vi "Dresden R2R Sputter 03.02.2018 IY24.vi"() -> ()   [LabVIEW 2009] (continued)
                        n14329 = while {
                          i -> [w20883]
                          stop <- w20884 stop-if-true
                          n14330 = Greater?(x=w20883, y=50) -> (0:w20881:bool)
                          n14331 = local read "Cnt_Left_slow_di"() -> (w20887:bool)
                          n14332 = case shown="True" w20881 {
                            frame #0 {
                            }
                            frame #1 {
                              n14333 = local write "Semi"(TRUE ("Semi")) -> ()
                              n14334 = local write "Error Message"("Transfer process was\ncancelled.Please check left slow sensor." ("Error Message")) -> ()
                            }
                          }
                          n14335 = case shown="False" w20887 {
                            tunnel: [FALSE ("Ch1_pet_cool_up_do") TRUE ("Ch1_pet_cool_up_do")] -> w20886
                            frame #0 {
                              n14336 = Wait Until Next ms Multiple(millisecond multiple=u32 200) -> ()  [unwired: 1 out]
                              n14337 = local write "Cnt_Left_slow_do"(TRUE ("Ch1_pet_cool_up_do")) -> ()
                            }
                            frame #1 {
                            }
                          }
                          n14338 = local read "Semi"() -> (w20885:bool)
                          n14339 = Or(x=w20886, y=w20885) -> (x .or. y?=w20884:bool)
                        }
                      }
                      frame #1 {
                      }
                    }
                  }
                  frame #3 {
                    n14340 = local read "Semi"() -> (w20894:bool)
                    n14341 = case shown="False" w20894 {
                      frame #0 {
                        n14342 = while {
                          i -> [w20897]
                          stop <- w20898 stop-if-true
                          n14343 = Greater?(x=w20897, y=50) -> (0:w20895:bool)
                          n14344 = local read "Cnt_Left_limit_di"() -> (w20901:bool)
                          n14345 = case shown="True" w20895 {
                            frame #0 {
                            }
                            frame #1 {
                              n14346 = local write "Semi"(TRUE ("Semi")) -> ()
                              n14347 = local write "Error Message"("Transfer process was\ncancelled.Please check left limit sensor." ("Error Message")) -> ()
                            }
                          }
                          n14348 = case shown="False" w20901 {
                            tunnel: [FALSE ("Ch1_pet_cool_up_do") TRUE ("Ch1_pet_cool_up_do")] -> w20900
                            frame #0 {
                              n14349 = Wait Until Next ms Multiple(millisecond multiple=u32 200) -> ()  [unwired: 1 out]
                              n14350 = local write "Cnt_Left_limit_do"(TRUE ("Ch1_pet_cool_up_do")) -> ()
                            }
                            frame #1 {
                            }
                          }
                          n14351 = local read "Semi"() -> (w20899:bool)
                          n14352 = Or(x=w20900, y=w20899) -> (x .or. y?=w20898:bool)
                        }
                      }
                      frame #1 {
                      }
                    }
                  }
                  frame #4 {
                    n14353 = local read "Semi"() -> (w20908:bool)
                    n14354 = case shown="False" w20908 {
                      frame #0 {
                        n14355 = local write "CH1_2trns_18"(TRUE ("CH1_2trns_7")) -> ()
                        n14356 = Wait (ms)(milliseconds to wait=u32 500) -> ()  [unwired: 1 out]
                      }
                      frame #1 {
                      }
                    }
                  }
                }
              }
              frame #1 {
              }
            }
          }
          frame #20 {
            n14357 = local read "Semi"() -> (w20911:bool)
            n14358 = case shown="False" w20911 {
              frame #0 {
                n14359 = local write "CH1_2trns_19"(TRUE ("CH1_2trns_18")) -> ()
                n14360 = local write "Cnt_Do_Buzzer"(TRUE ("Transfer_ch1_2")) -> ()
                n14361 = Wait (ms)(milliseconds to wait=u32 1500) -> ()  [unwired: 1 out]
              }
              frame #1 {
              }
            }
          }
          frame #21 {
            n14362 = local read "Semi"() -> (w20915:bool)
            n14363 = case shown="False" w20915 {
              frame #0 {
                n14364 = local write "ch_present_position"(4.0 ("ch_present_position")) -> ()
                n14365 = local write "Transfer_ch3_4"(FALSE ("Transfer_ch1_2")) -> ()
                n14366 = local write "Cnt_Do_Buzzer"(FALSE ("Transfer_ch1_2")) -> ()
                n14367 = Wait (ms)(milliseconds to wait=u32 500) -> ()  [unwired: 1 out]
              }
              frame #1 {
              }
            }
          }
        }
      }
      frame #6 {
        n14368 = stacked-sequence {
          frame #0 {
            n14369 = Wait (ms)(milliseconds to wait=u32 1500) -> ()  [unwired: 1 out]
            n14370 = local write "Clean_trnsfr_4_3"(TRUE ("Clean_trnsfr_1_2")) -> ()
            n14371 = local write "system_status"("Chamber 4 to Chamber 3 Transfer Process in Progress." ("system_status")) -> ()
            n14372 = local write "final_process_messages"("Chamber 4 to Chamber 3  Transfer Process was completed." ("final_process_messages")) -> ()
          }
          frame #1 {
            n14373 = stacked-sequence {
              frame #0 {
                n14374 = local write "Routine_check_transfer"(TRUE ("Routine_check_transfer")) -> ()
                n14375 = Wait (ms)(milliseconds to wait=u32 100) -> ()  [unwired: 1 out]
              }
              frame #1 {
                n14376 = while {
                  i -> [w20933]
                  stop <- w20929 stop-if-true
                  n14377 = Greater Or Equal?(x=w20933, y=1500) -> (x >= y?=w20930:bool)
                  n14378 = Wait Until Next ms Multiple(millisecond multiple=u32 200) -> ()  [unwired: 1 out]
                  n14379 = case shown="True" w20930 {
                    frame #0 {
                    }
                    frame #1 {
                      # "Hata mesajı"
                      n14380 = local write "Semi"(TRUE ("Semi")) -> ()
                    }
                  }
                  n14381 = local read "Routine_check_transfer"() -> (w20926:bool)
                  n14382 = local read "Semi"() -> (w20928:bool)
                  n14383 = Not(x=w20926) -> (.not. x?=w20927:bool)
                  n14384 = Or(x=w20927, y=w20928) -> (x .or. y?=w20929:bool)
                }
              }
              frame #2 {
                n14385 = Wait (ms)(milliseconds to wait=u32 500) -> ()  [unwired: 1 out]
              }
            }
          }
          frame #2 {
            # "STARTED UP CH3"
            n14386 = disable-structure shown="Disabled" {
              frame #0 {
                n14387 = local read "Semi"() -> (w20936:bool)
                n14388 = case shown="False" w20936 {
                  frame #0 {
                    n14389 = local read "started_up_ch3"() -> (w20937:bool)
                    n14390 = case shown="False" w20937 {
                      frame #0 {
                        n14391 = stacked-sequence {
                          frame #0 {
                            n14392 = local read "Semi"() -> (w20938:bool)
                            n14393 = case shown="False" w20938 {
                              frame #0 {
                                n14394 = local write "Start_up_ch3"(TRUE ("Start_up_ch2")) -> ()
                              }
                              frame #1 {
                              }
                            }
                          }
                          frame #1 {
                            n14395 = local read "Semi"() -> (w20940:bool)
                            n14396 = case shown="False" w20940 {
                              frame #0 {
                                n14397 = Wait (ms)(milliseconds to wait=u32 16000) -> ()  [unwired: 1 out]
                              }
                              frame #1 {
                              }
                            }
                          }
                          frame #2 {
                            n14398 = local read "Semi"() -> (w20942:bool)
                            n14399 = case shown="False" w20942 {
                              frame #0 {
                                n14400 = while {
                                i -> [w20947]
                                stop <- w20944 stop-if-true
                                n14401 = Greater?(x=w20947, y=80) -> (0:w20945:bool)
                                n14402 = local read "started_up_ch3"() -> (w20943:bool)
                                n14403 = case shown="True" w20945 {
                                frame #0 {
                                }
                                frame #1 {
                                n14404 = local write "Semi"(TRUE ("Semi")) -> ()
                                n14405 = local write "Error Message"("Chamber 1 Pressure is not suitable  \nfor transfer process!\nPlease check connections." ("Error Message")) -> ()
                                }
                                }
                                n14406 = case shown="False" w20943 {
                                tunnel: [FALSE TRUE] -> w20944
                                frame #0 {
                                n14407 = Wait Until Next ms Multiple(millisecond multiple=u32 200) -> ()  [unwired: 1 out]
                                }
                                frame #1 {
                                }
                                }
                                }
                              }
                              frame #1 {
                              }
                            }
                          }
                          frame #3 {
                            n14408 = local read "Semi"() -> (w20953:bool)
                            n14409 = case shown="False" w20953 {
                              frame #0 {
                                n14410 = local write "CH1_2_trns_0"(TRUE ("CH1_2_trns_0")) -> ()
                                n14411 = Wait (ms)(milliseconds to wait=u32 1000) -> ()  [unwired: 1 out]
                              }
                              frame #1 {
                              }
                            }
                          }
                        }
                      }
                      frame #1 {
                      }
                    }
                  }
                  frame #1 {
                  }
                }
              }
              frame #1 {
              }
            }
          }
          frame #3 {
            # "STARTED UP CH2"
            n14412 = disable-structure shown="Disabled" {
              frame #0 {
                n14413 = local read "Semi"() -> (w20956:bool)
                n14414 = case shown="False" w20956 {
                  frame #0 {
                    n14415 = local read "started_up_ch2"() -> (w20957:bool)
                    n14416 = case shown="False" w20957 {
                      frame #0 {
                        n14417 = stacked-sequence {
                          frame #0 {
                            n14418 = local read "Semi"() -> (w20958:bool)
                            n14419 = case shown="False" w20958 {
                              frame #0 {
                                n14420 = local write "Start_up_ch2"(TRUE ("Start_up_ch2")) -> ()
                              }
                              frame #1 {
                              }
                            }
                          }
                          frame #1 {
                            n14421 = local read "Semi"() -> (w20960:bool)
                            n14422 = case shown="False" w20960 {
                              frame #0 {
                                n14423 = Wait (ms)(milliseconds to wait=u32 18000) -> ()  [unwired: 1 out]
                              }
                              frame #1 {
                              }
                            }
                          }
                          frame #2 {
                            n14424 = local read "Semi"() -> (w20962:bool)
                            n14425 = case shown="False" w20962 {
                              frame #0 {
                                n14426 = while {
                                i -> [w20967]
                                stop <- w20964 stop-if-true
                                n14427 = Greater?(x=w20967, y=90) -> (0:w20965:bool)
                                n14428 = local read "started_up_ch2"() -> (w20963:bool)
                                n14429 = case shown="True" w20965 {
                                frame #0 {
                                }
                                frame #1 {
                                n14430 = local write "Semi"(TRUE ("Semi")) -> ()
                                n14431 = local write "Error Message"("Chamber 2 Pressure is not suitable  \nfor transfer process!\nPlease check connections." ("Error Message")) -> ()
                                }
                                }
                                n14432 = case shown="False" w20963 {
                                tunnel: [FALSE TRUE] -> w20964
                                frame #0 {
                                n14433 = Wait Until Next ms Multiple(millisecond multiple=u32 200) -> ()  [unwired: 1 out]
                                }
                                frame #1 {
                                }
                                }
                                }
                              }
                              frame #1 {
                              }
                            }
                          }
                          frame #3 {
                            n14434 = local read "Semi"() -> (w20973:bool)
                            n14435 = case shown="False" w20973 {
                              frame #0 {
                                n14436 = local write "CH1_2_trns_1"(TRUE ("CH1_2_trns_0")) -> ()
                                n14437 = Wait (ms)(milliseconds to wait=u32 1000) -> ()  [unwired: 1 out]
                              }
                              frame #1 {
                              }
                            }
                          }
                        }
                      }
                      frame #1 {
                      }
                    }
                  }
                  frame #1 {
                  }
                }
              }
              frame #1 {
              }
            }
          }
          frame #4 {
            # "TRNS GV-BP OPEN"
            n14438 = local read "Semi"() -> (w20976:bool)
            n14439 = case shown="False" w20976 {
              frame #0 {
                n14440 = stacked-sequence {
                  frame #0 {
                    n14441 = local read "Semi"() -> (w20977:bool)
                    n14442 = case shown="False" w20977 {
                      frame #0 {
                        n14443 = while {
                          i -> [w20984]
                          stop <- w20979 stop-if-true
                          n14444 = Greater?(x=w20984, y=50) -> (0:w20982:bool)
                          n14445 = local read "Ch3_Trns_gv_bp2_di"() -> (w20978:bool)
                          n14446 = case shown="True" w20982 {
                            frame #0 {
                            }
                            frame #1 {
                              n14447 = local write "Semi"(TRUE ("Semi")) -> ()
                              n14448 = local write "Error Message"("Transfer process was cancelled.\nPlease check CH1-Trns-GV connections." ("Error Message")) -> ()
                            }
                          }
                          n14449 = case shown="False" w20978 {
                            tunnel: [FALSE TRUE] -> w20981
                            frame #0 {
                              n14450 = Wait Until Next ms Multiple(millisecond multiple=u32 200) -> ()  [unwired: 1 out]
                              n14451 = local write "Ch3_Trns_gv_bp2_do"(TRUE ("Ch1_pet_cool_up_do")) -> ()
                            }
                            frame #1 {
                            }
                          }
                          n14452 = local read "Semi"() -> (w20980:bool)
                          n14453 = Or(x=w20981, y=w20980) -> (x .or. y?=w20979:bool)
                        }
                      }
                      frame #1 {
                      }
                    }
                  }
                  frame #1 {
                    n14454 = local read "Semi"() -> (w20991:bool)
                    n14455 = case shown="False" w20991 {
                      frame #0 {
                        n14456 = Wait (ms)(milliseconds to wait=u32 500) -> ()  [unwired: 1 out]
                      }
                      frame #1 {
                      }
                    }
                  }
                  frame #2 {
                    n14457 = local read "Semi"() -> (w20993:bool)
                    n14458 = case shown="False" w20993 {
                      frame #0 {
                        n14459 = while {
                          i -> [w21000]
                          stop <- w20995 stop-if-true
                          n14460 = Greater?(x=w21000, y=50) -> (0:w20998:bool)
                          n14461 = local read "Ch4_Trns_gv_bp_di"() -> (w20994:bool)
                          n14462 = case shown="True" w20998 {
                            frame #0 {
                            }
                            frame #1 {
                              n14463 = local write "Semi"(TRUE ("Semi")) -> ()
                              n14464 = local write "Error Message"("Transfer process was cancelled.\nPlease check CH1-Trns-GV connections." ("Error Message")) -> ()
                            }
                          }
                          n14465 = case shown="False" w20994 {
                            tunnel: [FALSE TRUE] -> w20997
                            frame #0 {
                              n14466 = local write "Ch4_Trns_gv_bp_do"(TRUE ("Ch1_pet_cool_up_do")) -> ()
                              n14467 = Wait Until Next ms Multiple(millisecond multiple=u32 200) -> ()  [unwired: 1 out]
                            }
                            frame #1 {
                            }
                          }
                          n14468 = local read "Semi"() -> (w20996:bool)
                          n14469 = Or(x=w20997, y=w20996) -> (x .or. y?=w20995:bool)
                        }
                      }
                      frame #1 {
                      }
                    }
                  }
                  frame #3 {
                    n14470 = local read "Semi"() -> (w21007:bool)
                    n14471 = case shown="False" w21007 {
                      frame #0 {
                        n14472 = Wait (ms)(milliseconds to wait=u32 500) -> ()  [unwired: 1 out]
                      }
                      frame #1 {
                      }
                    }
                  }
                }
              }
              frame #1 {
              }
            }
          }
          frame #5 {
            # "TRNS GV OPEN"
            n14473 = local read "Semi"() -> (w21009:bool)
            n14474 = case shown="False" w21009 {
              frame #0 {
                n14475 = stacked-sequence {
                  frame #0 {
                    n14476 = local read "Semi"() -> (w21010:bool)
                    n14477 = case shown="False" w21010 {
                      frame #0 {
                        n14478 = local write "Ch3_Trns_gv_close_do"(FALSE ("Ch1_pet_cool_up_do")) -> ()
                      }
                      frame #1 {
                      }
                    }
                  }
                  frame #1 {
                    n14479 = local read "Semi"() -> (w21012:bool)
                    n14480 = case shown="False" w21012 {
                      frame #0 {
                        n14481 = while {
                          i -> [w21019]
                          stop <- w21014 stop-if-true
                          n14482 = Greater?(x=w21019, y=500) -> (0:w21017:bool)
                          n14483 = local read "Ch3_Trns_gv_open_di"() -> (w21013:bool)
                          n14484 = case shown="True" w21017 {
                            frame #0 {
                            }
                            frame #1 {
                              n14485 = local write "Semi"(TRUE ("Semi")) -> ()
                              n14486 = local write "Error Message"("Transfer process was cancelled.\nPlease check CH1-Trns-GV connections." ("Error Message")) -> ()
                            }
                          }
                          n14487 = case shown="False" w21013 {
                            tunnel: [FALSE TRUE] -> w21016
                            frame #0 {
                              n14488 = Wait Until Next ms Multiple(millisecond multiple=u32 200) -> ()  [unwired: 1 out]
                              n14489 = local write "Ch3_Trns_gv_open_do"(TRUE ("Ch1_pet_cool_up_do")) -> ()
                            }
                            frame #1 {
                            }
                          }
                          n14490 = local read "Semi"() -> (w21015:bool)
                          n14491 = Or(x=w21016, y=w21015) -> (x .or. y?=w21014:bool)
                        }
                      }
                      frame #1 {
                      }
                    }
                  }
                  frame #2 {
                    n14492 = local read "Semi"() -> (w21026:bool)
                    n14493 = case shown="False" w21026 {
                      frame #0 {
                        n14494 = local write "CH1_2trns_2"(TRUE ("CH1_2trns_5")) -> ()
                        n14495 = Wait (ms)(milliseconds to wait=u32 500) -> ()  [unwired: 1 out]
                      }
                      frame #1 {
                      }
                    }
                  }
                }
              }
              frame #1 {
              }
            }
          }
          frame #6 {
            # "TRNS GV control Trnsgv 2_3"
            n14496 = local read "Semi"() -> (w21029:bool)
            n14497 = case shown="False" w21029 {
              frame #0 {
                n14498 = stacked-sequence {
                  frame #0 {
                    n14499 = local read "Semi"() -> (w21030:bool)
                    n14500 = case shown="False" w21030 {
                      frame #0 {
                        n14501 = while {
                          i -> [w21037]
                          stop <- w21032 stop-if-true
                          n14502 = Greater?(x=w21037, y=50) -> (0:w21035:bool)
                          n14503 = local read "Ch3_TGV_control_di"() -> (w21031:bool)
                          n14504 = case shown="True" w21035 {
                            frame #0 {
                            }
                            frame #1 {
                              n14505 = local write "Semi"(TRUE ("Semi")) -> ()
                              n14506 = local write "Error Message"("Transfer process was cancelled.\nPlease check TRNS-GV connections." ("Error Message")) -> ()
                            }
                          }
                          n14507 = case shown="True" w21031 {
                            tunnel: [TRUE FALSE] -> w21034
                            frame #0 {
                            }
                            frame #1 {
                              n14508 = Wait Until Next ms Multiple(millisecond multiple=u32 200) -> ()  [unwired: 1 out]
                              n14509 = local write "Ch3_TGV_control_do"(FALSE ("Ch1_pet_cool_up_do")) -> ()
                            }
                          }
                          n14510 = local read "Semi"() -> (w21033:bool)
                          n14511 = Or(x=w21034, y=w21033) -> (x .or. y?=w21032:bool)
                        }
                      }
                      frame #1 {
                      }
                    }
                  }
                  frame #1 {
                    n14512 = local read "Semi"() -> (w21044:bool)
                    n14513 = case shown="False" w21044 {
                      frame #0 {
                        n14514 = local write "CH1_2trns_3"(TRUE ("CH1_2trns_5")) -> ()
                        n14515 = Wait (ms)(milliseconds to wait=u32 500) -> ()  [unwired: 1 out]
                      }
                      frame #1 {
                      }
                    }
                  }
                }
              }
              frame #1 {
              }
            }
          }
          frame #7 {
            # "TRNS GV control Trnsgv 2_3"
            n14516 = local read "Semi"() -> (w21047:bool)
            n14517 = case shown="False" w21047 {
              frame #0 {
                n14518 = stacked-sequence {
                  frame #0 {
                    n14519 = local read "Semi"() -> (w21048:bool)
                    n14520 = case shown="False" w21048 {
                      frame #0 {
                        n14521 = while {
                          i -> [w21055]
                          stop <- w21050 stop-if-true
                          n14522 = Greater?(x=w21055, y=50) -> (0:w21053:bool)
                          n14523 = local read "Ch1_Trns_interlock_di"() -> (w21049:bool)
                          n14524 = case shown="True" w21053 {
                            frame #0 {
                            }
                            frame #1 {
                              n14525 = local write "Semi"(TRUE ("Semi")) -> ()
                              n14526 = local write "Error Message"("Transfer process was cancelled.\nPlease check TRNS-GV connections." ("Error Message")) -> ()
                            }
                          }
                          n14527 = case shown="False" w21049 {
                            tunnel: [w21057 TRUE] -> w21052
                            frame #0 {
                              n14528 = local read "Ch1_TGV_control_di"() -> (w21056:bool)
                              n14529 = case shown="False" w21056 {
                                tunnel: [FALSE TRUE] -> w21057
                                frame #0 {
                                n14530 = Wait Until Next ms Multiple(millisecond multiple=u32 200) -> ()  [unwired: 1 out]
                                n14531 = local write "Ch1_TGV_control_do"(TRUE ("Ch1_pet_cool_up_do")) -> ()
                                }
                                frame #1 {
                                }
                              }
                            }
                            frame #1 {
                            }
                          }
                          n14532 = local read "Semi"() -> (w21051:bool)
                          n14533 = Or(x=w21052, y=w21051) -> (x .or. y?=w21050:bool)
                        }
                      }
                      frame #1 {
                      }
                    }
                  }
                  frame #1 {
                    n14534 = local read "Semi"() -> (w21065:bool)
                    n14535 = case shown="False" w21065 {
                      frame #0 {
                        n14536 = local write "CH1_2trns_3"(TRUE ("CH1_2trns_5")) -> ()
                        n14537 = Wait (ms)(milliseconds to wait=u32 500) -> ()  [unwired: 1 out]
                      }
                      frame #1 {
                      }
                    }
                  }
                }
              }
              frame #1 {
              }
            }
          }
          frame #8 {
            # "TRNS GV control Trnsgv 3_4"
            n14538 = local read "Semi"() -> (w21068:bool)
            n14539 = case shown="False" w21068 {
              frame #0 {
                n14540 = stacked-sequence {
                  frame #0 {
                    n14541 = local read "Semi"() -> (w21069:bool)
                    n14542 = case shown="False" w21069 {
                      frame #0 {
                        n14543 = while {
                          i -> [w21076]
                          stop <- w21071 stop-if-true
                          n14544 = Greater?(x=w21076, y=50) -> (0:w21074:bool)
                          n14545 = local read "Ch2_Trns_interlock_di"() -> (w21070:bool)
                          n14546 = case shown="True" w21074 {
                            frame #0 {
                            }
                            frame #1 {
                              n14547 = local write "Semi"(TRUE ("Semi")) -> ()
                              n14548 = local write "Error Message"("Transfer process was cancelled.\nPlease check TRNS-GV connections." ("Error Message")) -> ()
                            }
                          }
                          n14549 = case shown="False" w21070 {
                            tunnel: [w21078 TRUE] -> w21073
                            frame #0 {
                              n14550 = local read "Ch2_TGV_control_di"() -> (w21077:bool)
                              n14551 = case shown="False" w21077 {
                                tunnel: [FALSE TRUE] -> w21078
                                frame #0 {
                                n14552 = Wait Until Next ms Multiple(millisecond multiple=u32 200) -> ()  [unwired: 1 out]
                                n14553 = local write "Ch2_TGV_control_do"(TRUE ("Ch1_pet_cool_up_do")) -> ()
                                }
                                frame #1 {
                                }
                              }
                            }
                            frame #1 {
                            }
                          }
                          n14554 = local read "Semi"() -> (w21072:bool)
                          n14555 = Or(x=w21073, y=w21072) -> (x .or. y?=w21071:bool)
                        }
                      }
                      frame #1 {
                      }
                    }
                  }
                  frame #1 {
                    n14556 = local read "Semi"() -> (w21086:bool)
                    n14557 = case shown="False" w21086 {
                      frame #0 {
                        n14558 = local write "CH1_2trns_4"(TRUE ("CH1_2trns_5")) -> ()
                        n14559 = Wait (ms)(milliseconds to wait=u32 500) -> ()  [unwired: 1 out]
                      }
                      frame #1 {
                      }
                    }
                  }
                }
              }
              frame #1 {
              }
            }
          }
          frame #9 {
            # "Left slow deactive"
            n14560 = local read "Semi"() -> (w21089:bool)
            n14561 = case shown="False" w21089 {
              frame #0 {
                n14562 = stacked-sequence {
                  frame #0 {
                    n14563 = local read "Semi"() -> (w21090:bool)
                    n14564 = case shown="False" w21090 {
                      frame #0 {
                        n14565 = while {
                          i -> [w21093]
                          stop <- w21094 stop-if-true
                          n14566 = Greater?(x=w21093, y=50) -> (0:w21091:bool)
                          n14567 = local read "Cnt_Left_slow_di"() -> (w21097:bool)
                          n14568 = case shown="True" w21091 {
                            frame #0 {
                            }
                            frame #1 {
                              n14569 = local write "Semi"(TRUE ("Semi")) -> ()
                              n14570 = local write "Error Message"("Transfer process was\ncancelled.Please check right slow sensor." ("Error Message")) -> ()
                            }
                          }
                          n14571 = case shown="True" w21097 {
                            tunnel: [FALSE ("Ch1_pet_cool_up_do") TRUE ("Ch1_pet_cool_up_do")] -> w21096
                            frame #0 {
                              n14572 = Wait Until Next ms Multiple(millisecond multiple=u32 200) -> ()  [unwired: 1 out]
                              n14573 = local write "Cnt_Left_slow_do"(TRUE ("Ch1_pet_cool_up_do")) -> ()
                            }
                            frame #1 {
                            }
                          }
                          n14574 = local read "Semi"() -> (w21095:bool)
                          n14575 = Or(x=w21096, y=w21095) -> (x .or. y?=w21094:bool)
                        }
                      }
                      frame #1 {
                      }
                    }
                  }
                  frame #1 {
                    n14576 = local read "Semi"() -> (w21104:bool)
                    n14577 = case shown="False" w21104 {
                      frame #0 {
                        n14578 = local write "CH1_2trns_5"(TRUE ("CH1_2trns_7")) -> ()
                        n14579 = Wait (ms)(milliseconds to wait=u32 500) -> ()  [unwired: 1 out]
                      }
                      frame #1 {
                      }
                    }
                  }
                }
              }
              frame #1 {
              }
            }
          }
          frame #10 {
            # "Left limit deactive"
            n14580 = local read "Semi"() -> (w21107:bool)
            n14581 = case shown="False" w21107 {
              frame #0 {
                n14582 = stacked-sequence {
                  frame #0 {
                    n14583 = local read "Semi"() -> (w21108:bool)
                    n14584 = case shown="False" w21108 {
                      frame #0 {
                        n14585 = while {
                          i -> [w21109]
                          stop <- w21113 stop-if-true
                          n14586 = Greater?(x=w21109, y=50) -> (0:w21111:bool)
                          n14587 = local read "Cnt_Left_limit_di"() -> (w21115:bool)
                          n14588 = case shown="True" w21111 {
                            frame #0 {
                            }
                            frame #1 {
                              n14589 = local write "Semi"(TRUE ("Semi")) -> ()
                              n14590 = local write "Error Message"("Transfer process was\ncancelled.Please check right limit sensor." ("Error Message")) -> ()
                            }
                          }
                          n14591 = case shown="True" w21115 {
                            tunnel: [FALSE ("Ch1_pet_cool_up_do") TRUE ("Ch1_pet_cool_up_do")] -> w21114
                            frame #0 {
                              n14592 = Wait Until Next ms Multiple(millisecond multiple=u32 200) -> ()  [unwired: 1 out]
                              n14593 = local write "Cnt_Left_limit_do"(TRUE ("Ch1_pet_cool_up_do")) -> ()
                            }
                            frame #1 {
                            }
                          }
                          n14594 = local read "Semi"() -> (w21112:bool)
                          n14595 = Or(x=w21114, y=w21112) -> (x .or. y?=w21113:bool)
                        }
                      }
                      frame #1 {
                      }
                    }
                  }
                  frame #1 {
                    n14596 = local read "Semi"() -> (w21122:bool)
                    n14597 = case shown="False" w21122 {
                      frame #0 {
                        n14598 = local write "CH1_2trns_6"(TRUE ("CH1_2trns_7")) -> ()
                        n14599 = Wait (ms)(milliseconds to wait=u32 500) -> ()  [unwired: 1 out]
                      }
                      frame #1 {
                      }
                    }
                  }
                }
              }
              frame #1 {
              }
            }
          }
          frame #11 {
            # "Right slow active"
            n14600 = local read "Semi"() -> (w21125:bool)
            n14601 = case shown="False" w21125 {
              frame #0 {
                n14602 = stacked-sequence {
                  frame #0 {
                    n14603 = local read "Semi"() -> (w21126:bool)
                    n14604 = case shown="False" w21126 {
                      frame #0 {
                        n14605 = while {
                          i -> [w21127]
                          stop <- w21131 stop-if-true
                          n14606 = Greater?(x=w21127, y=50) -> (0:w21129:bool)
                          n14607 = local read "Cnt_Right_slow_di"() -> (w21133:bool)
                          n14608 = case shown="True" w21129 {
                            frame #0 {
                            }
                            frame #1 {
                              n14609 = local write "Semi"(TRUE ("Semi")) -> ()
                              n14610 = local write "Error Message"("Transfer process was\ncancelled.Please check left slow sensor." ("Error Message")) -> ()
                            }
                          }
                          n14611 = case shown="True" w21133 {
                            tunnel: [TRUE ("Ch1_pet_cool_up_do") FALSE ("Ch1_pet_cool_up_do")] -> w21132
                            frame #0 {
                            }
                            frame #1 {
                              n14612 = local write "Cnt_Right_slow_do"(FALSE ("Ch1_pet_cool_up_do")) -> ()
                              n14613 = Wait Until Next ms Multiple(millisecond multiple=u32 200) -> ()  [unwired: 1 out]
                            }
                          }
                          n14614 = local read "Semi"() -> (w21130:bool)
                          n14615 = Or(x=w21132, y=w21130) -> (x .or. y?=w21131:bool)
                        }
                      }
                      frame #1 {
                      }
                    }
                  }
                  frame #1 {
                    n14616 = local read "Semi"() -> (w21140:bool)
                    n14617 = case shown="False" w21140 {
                      frame #0 {
                        n14618 = local write "CH1_2trns_7"(TRUE ("CH1_2trns_6b")) -> ()
                        n14619 = Wait (ms)(milliseconds to wait=u32 500) -> ()  [unwired: 1 out]
                      }
                      frame #1 {
                      }
                    }
                  }
                }
              }
              frame #1 {
              }
            }
          }
          frame #12 {
            # "Right limit active"
            n14620 = local read "Semi"() -> (w21143:bool)
            n14621 = case shown="False" w21143 {
              frame #0 {
                n14622 = stacked-sequence {
                  frame #0 {
                    n14623 = local read "Semi"() -> (w21144:bool)
                    n14624 = case shown="False" w21144 {
                      frame #0 {
                        n14625 = while {
                          i -> [w21145]
                          stop <- w21149 stop-if-true
                          n14626 = Greater?(x=w21145, y=50) -> (0:w21147:bool)
                          n14627 = local read "Cnt_Right_limit_di"() -> (w21151:bool)
                          n14628 = case shown="True" w21147 {
                            frame #0 {
                            }
                            frame #1 {
                              n14629 = local write "Semi"(TRUE ("Semi")) -> ()
                              n14630 = local write "Error Message"("Transfer process was\ncancelled.Please check left limit sensor." ("Error Message")) -> ()
                            }
                          }
                          n14631 = case shown="True" w21151 {
                            tunnel: [TRUE ("Ch1_pet_cool_up_do") FALSE ("Ch1_pet_cool_up_do")] -> w21150
                            frame #0 {
                            }
                            frame #1 {
                              n14632 = local write "Cnt_Right_limit_do"(FALSE ("Ch1_pet_cool_up_do")) -> ()
                              n14633 = Wait Until Next ms Multiple(millisecond multiple=u32 200) -> ()  [unwired: 1 out]
                            }
                          }
                          n14634 = local read "Semi"() -> (w21148:bool)
                          n14635 = Or(x=w21150, y=w21148) -> (x .or. y?=w21149:bool)
                        }
                      }
                      frame #1 {
                      }
                    }
                  }
                  frame #1 {
                    n14636 = local read "Semi"() -> (w21158:bool)
                    n14637 = case shown="False" w21158 {
                      frame #0 {
                        n14638 = local write "CH1_2trns_8"(TRUE ("CH1_2trns_6c")) -> ()
                        n14639 = Wait (ms)(milliseconds to wait=u32 500) -> ()  [unwired: 1 out]
                      }
                      frame #1 {
                      }
                    }
                  }
                }
              }
              frame #1 {
              }
            }
          }
          frame #13 {
            # "Casette Direction"
            n14640 = local read "Semi"() -> (w21161:bool)
            n14641 = case shown="False" w21161 {
              frame #0 {
                n14642 = stacked-sequence {
                  frame #0 {
                    n14643 = local read "Semi"() -> (w21162:bool)
                    n14644 = case shown="False" w21162 {
                      frame #0 {
                        n14645 = while {
                          i -> [w21168]
                          stop <- w21163 stop-if-true
                          n14646 = Greater?(x=w21168, y=50) -> (0:w21169:bool)
                          n14647 = case shown="True" w21169 {
                            frame #0 {
                            }
                            frame #1 {
                              n14648 = local write "Semi"(TRUE ("Semi")) -> ()
                              n14649 = local write "Error Message"("Transfer process was cancelled.\nPlease check Casette Direction connections." ("Error Message")) -> ()
                            }
                          }
                          n14650 = local read "Casette_servo_left_direction_di"() -> (w21166:bool)
                          n14651 = case shown="True" w21166 {
                            tunnel: [TRUE ("Casette_servo_left_direction_do") FALSE ("Casette_servo_left_direction_do")] -> w21165
                            frame #0 {
                            }
                            frame #1 {
                              n14652 = Wait Until Next ms Multiple(millisecond multiple=u32 200) -> ()  [unwired: 1 out]
                              n14653 = local write "Casette_servo_left_direction_do"(FALSE ("Casette_servo_left_direction_do")) -> ()
                            }
                          }
                          n14654 = local read "Semi"() -> (w21164:bool)
                          n14655 = Or(x=w21165, y=w21164) -> (x .or. y?=w21163:bool)
                        }
                      }
                      frame #1 {
                      }
                    }
                  }
                  frame #1 {
                    n14656 = local read "Semi"() -> (w21176:bool)
                    n14657 = case shown="False" w21176 {
                      frame #0 {
                        n14658 = local write "CH1_2trns_9"(TRUE ("CH1_2trns_7")) -> ()
                        n14659 = Wait (ms)(milliseconds to wait=u32 500) -> ()  [unwired: 1 out]
                      }
                      frame #1 {
                      }
                    }
                  }
                }
              }
              frame #1 {
              }
            }
          }
          frame #14 {
            # "SET CASSETTE SERVO  SPEED 300"
            n14660 = local read "Semi"() -> (w21179:bool)
            n14661 = case shown="False" w21179 {
              frame #0 {
                n14662 = stacked-sequence {
                  frame #0 {